vi "HFRR ADV v043.vi"() -> ()   [LabVIEW 2025] (continued)
            n814 = Subtract(x=w847, y=w851) -> (x-y=w855:dbl)
            n815 = In Range and Coerce(upper limit=w858, x=w850, lower limit=w857) -> (In Range?=w854:bool)  [unwired: 1 out]
            n816 = In Range and Coerce(upper limit=w856, x=w849, lower limit=w855) -> (In Range?=w853:bool)  [unwired: 1 out]
            n817 = And(x=w854, y=w853) -> (x .and. y?=w852:bool)
            n818 = case shown="True" w852 {
              frame False {
                n819 = property on="Accept & Save Air Temperature step 4" class="Bool (strict)"("DisabledEnum"=T19."Disabled" ("Disabled")) -> ()  [unwired: 2 in, 2 out]
                n820 = local write "Air Temperature Calibration"(enum32{"True", "Fail"}."Fail" ("Sample Temperature Calibration  2")) -> ()
              }
              frame True {
                n821 = local write "Air Temperature Calibration"(enum32{"True", "Fail"}."True" ("Sample Temperature Calibration  2")) -> ()
                n822 = property on="Accept & Save Air Temperature step 4" class="Bool (strict)"("DisabledEnum"=T19."Enabled" ("Disabled")) -> ()  [unwired: 2 in, 2 out]
              }
            }
          }
          frame #8 {
            # "CAL;END"
          }
          frame #9 {
            n823 = local write "Tab Control 4"(T12."Air Step 4" ("Tab Control 4")) -> ()
          }
        }
      }
      event "Back Stroke step main temperature": Value Change {
        n824 = event-data() -> ()  [unwired: 1 in, 6 out]
        n825 = stacked-sequence {
          frame #0 {
            n826 = Wait (ms)(milliseconds to wait=u32 1000) -> ()  [unwired: 1 out]
          }
          frame #1 {
            # "CAL;END"
            n827 = local write "Due Write"("CAL;END" ("Command")) -> ()
          }
          frame #2 {
            n828 = Wait (ms)(milliseconds to wait=u32 1000) -> ()  [unwired: 1 out]
          }
          frame #3 {
            # "CAL;END"
            n829 = local write "Due Write"("CAL;END" ("Command")) -> ()
          }
          frame #4 {
            n830 = local write "Temperature Selection"(T13."Default" ("Temperature Selection")) -> ()
            n831 = local write "Calibration Selection"(T8."Default" ("Calibration Selection")) -> ()
            n832 = local write "Main Calibration Tab"(T7."Main" ("Main Calibration Tab")) -> ()
            n833 = local write "Tab Control 4"(T12."Main" ("Tab Control 4")) -> ()
          }
        }
      }
      event "TEMPERATURE STEP  Back 4", "TEMPERATURE STEP 1 Back 3", "TEMPERATURE STEP  Back 3", "TEMPERATURE STEP 1 Back 2", "Back Air TEMPERATURE Step 4", "Back SAMPLE TEMPERATURE Step 4": Value Change {
        # "Back Stroke step main temperature"
        n834 = event-data() -> ()  [unwired: 1 in, 6 out]
        n835 = stacked-sequence {
          frame #0 {
            n836 = Wait (ms)(milliseconds to wait=u32 1000) -> ()  [unwired: 1 out]
          }
          frame #1 {
            # "CAL;END"
            n837 = local write "Due Write"("CAL;END" ("Command")) -> ()
          }
          frame #2 {
            n838 = Wait (ms)(milliseconds to wait=u32 1000) -> ()  [unwired: 1 out]
          }
          frame #3 {
            # "CAL;END"
            n839 = local write "Due Write"("CAL;END" ("Command")) -> ()
          }
          frame #4 {
            # "TEMPERATURE STEP  Back 4"
            n840 = local write "Main Calibration Tab"(T7."Temperature" ("Main Calibration Tab")) -> ()
            n841 = local write "Temperature Selection"(T13."Default" ("Temperature Selection")) -> ()
            n842 = local write "Tab Control 4"(T12."Main" ("Tab Control 4")) -> ()
            n843 = local write "Calibration Selection"(T8."Default" ("Calibration Selection")) -> ()
          }
        }
      }
      event "FF BACK", "FF BACK 2", "FF BACK 3", "FF BACK 4", "FF BACK 5", "FF BACK 6": Value Change {
        n844 = event-data() -> ()  [unwired: 1 in, 6 out]
        n845 = stacked-sequence {
          frame #0 {
            n846 = Wait (ms)(milliseconds to wait=u32 1000) -> ()  [unwired: 1 out]
          }
          frame #1 {
            n847 = local write "Due Write"("VC;0") -> ()
          }
          frame #2 {
            n848 = Wait (ms)(milliseconds to wait=u32 1000) -> ()  [unwired: 1 out]
          }
          frame #3 {
            n849 = local write "Due Write"("VC;0") -> ()
          }
          frame #4 {
            w884 = FALSE
            n850 = local write "FF BACK 2"(w884) -> ()
            n851 = local write "FF BACK 3"(w884) -> ()
            n852 = local write "FF BACK 4"(w884) -> ()
            n853 = local write "FF BACK 5"(w884) -> ()
            n854 = local write "FF BACK 6"(w884) -> ()
            n855 = local write "FF BACK"(w884) -> ()
          }
          frame #5 {
            n856 = local write "Temperature Selection"(T13."Default" ("Temperature Selection")) -> ()
            n857 = local write "Calibration Selection"(T8."Default" ("Calibration Selection")) -> ()
            n858 = local write "Friction Force Tab"(T11."Page 1" ("Friction Force Tab")) -> ()
            n859 = local write "Main Calibration Tab"(T7."Main" ("Main Calibration Tab")) -> ()
            n860 = property on="Tab Control 6" class="TabCtl (strict)"("Visible"=FALSE) -> ()  [unwired: 2 in, 2 out]
            n861 = property on="Friction Force Calibration Result Tab" class="TabCtl (strict)"("Visible"=FALSE) -> ()  [unwired: 2 in, 2 out]
          }
        }
      }
      event "Accept & Save FF": Value Change {
        n862 = event-data() -> ()  [unwired: 1 in, 6 out]
        n863 = stacked-sequence {
          frame #0 {
            n864 = Wait (ms)(milliseconds to wait=u32 1000) -> ()  [unwired: 1 out]
          }
          frame #1 {
            n865 = local write "Due Write"("VC;0") -> ()
          }
          frame #2 {
            n866 = Wait (ms)(milliseconds to wait=u32 1000) -> ()  [unwired: 1 out]
          }
          frame #3 {
            n867 = local write "Due Write"("VC;0") -> ()
          }
          frame #4 {
            w895 = FALSE
            n868 = local write "FF BACK 2"(w895) -> ()
            n869 = local write "FF BACK 3"(w895) -> ()
            n870 = local write "FF BACK 4"(w895) -> ()
            n871 = local write "FF BACK 5"(w895) -> ()
            n872 = local write "FF BACK 6"(w895) -> ()
            n873 = local write "FF BACK"(w895) -> ()
          }
          frame #5 {
            n874 = Get Date/Time In Seconds() -> (seconds since 1Jan1904=w898:timestamp)
            n875 = Format Into String(format string="%<%I:%M:%S:%p %d:%B:%Y>T", w898) -> (resulting string=w896:string)  [unwired: 2 in, 1 out]
            n876 = local write "FRICTION CALIBRATION"(w896) -> ()
          }
          frame #6 {
            n877 = local write "Temperature Selection"(T13."Default" ("Temperature Selection")) -> ()
            n878 = local write "Calibration Selection"(T8."Default" ("Calibration Selection")) -> ()
            n879 = local write "Friction Force Tab"(T11."Page 1" ("Friction Force Tab")) -> ()
            n880 = local write "Main Calibration Tab"(T7."Main" ("Main Calibration Tab")) -> ()
            n881 = local write "Save Button"(TRUE ("Save Button")) -> ()
            n882 = property on="Tab Control 6" class="TabCtl (strict)"("Visible"=FALSE) -> ()  [unwired: 2 in, 2 out]
            n883 = property on="Friction Force Calibration Result Tab" class="TabCtl (strict)"("Visible"=FALSE) -> ()  [unwired: 2 in, 2 out]
          }
        }
      }
      event "FF CONTINUE": Value Change {
        n884 = event-data() -> ()  [unwired: 1 in, 6 out]
        n885 = local write "FF CONTINUE"(FALSE ("FF CONTINUE")) -> ()
        n886 = local write "Friction Force Tab"(T11."Page 2" ("Friction Force Tab")) -> ()
      }
      event "FF CONTINUE 2": Value Change {
        n887 = event-data() -> ()  [unwired: 1 in, 6 out]
        n888 = local write "FF CONTINUE 2"(FALSE ("FF CONTINUE")) -> ()
        n889 = local write "Friction Force Tab"(T11."Page 3" ("Friction Force Tab")) -> ()
      }
      event "FF CONTINUE 3": Value Change {
        n890 = event-data() -> ()  [unwired: 1 in, 6 out]
        n891 = local write "FF CONTINUE 3"(FALSE ("FF CONTINUE")) -> ()
        n892 = local write "Friction Force Tab"(T11."Page 4" ("Friction Force Tab")) -> ()
      }
      event "FF CONTINUE 4": Value Change {
        n893 = event-data() -> ()  [unwired: 1 in, 6 out]
        n894 = local write "FF CONTINUE 4"(FALSE ("FF CONTINUE")) -> ()
        n895 = local write "Friction Force Tab"(T11."Page 5" ("Friction Force Tab")) -> ()
        n896 = property on="Friction Force Calibration Result Tab" class="TabCtl (strict)"("Visible"=FALSE) -> ()  [unwired: 2 in, 2 out]
      }
      event "FF CONTINUE 5": Value Change {
        n897 = event-data() -> ()  [unwired: 1 in, 6 out]
        n898 = local write "FF CONTINUE 5"(FALSE ("FF CONTINUE")) -> ()
        n899 = local write "Friction Force Tab"(T11."Page 6" ("Friction Force Tab")) -> ()
        n900 = property on="Friction Force Calibration Result Tab" class="TabCtl (strict)"("Visible"=FALSE) -> ()  [unwired: 2 in, 2 out]
        n901 = property on="Tab Control 6" class="TabCtl (strict)"("Visible"=FALSE) -> ()  [unwired: 2 in, 2 out]
      }
      event "Stroke Report Button": Value Change {
        n902 = event-data() -> ()  [unwired: 1 in, 6 out]
        n903 = local read "Point 5 - 1.0 mm"() -> (w920:bool)
        n904 = case shown="False" w920 {
          tunnel: [0.8 1.0] -> w919
          frame False {
          }
          frame True {
          }
        }
        n905 = local read "Machine Serial Number"() -> (w923:string)
        n906 = local read "USERNAME"() -> (w921:string)
        n907 = local write "Stroke Report Button"(FALSE ("Stroke Report Button")) -> ()
        n908 = call "Stroke Calibration Report.vi"("measured_value"=w919, "operator_name"=w921, "Instrument_serial Number"=w923) -> ()  [unwired: 7 in, 2 out]
      }
      event "Sample Report Button": Value Change {
        n909 = event-data() -> ()  [unwired: 1 in, 6 out]
        n910 = local read "Machine Serial Number"() -> (w929:string)
        n911 = local read "Sample 0deg temp"() -> (w926:dbl)
        n912 = local read "Sample 60deg temp"() -> (w927:dbl)
        n913 = local read "USERNAME"() -> (w928:string)
        n914 = call "Temperature Calibration Report.vi"("measured_60"=w927, "measured_zero"=w926, "operator_name"=w928, "Instrument_serial Number"=w929) -> ()  [unwired: 6 in, 2 out]
        n915 = local write "Sample Report Button"(FALSE ("Sample Report Button")) -> ()
      }
      event "Report Button FF": Value Change {
        n916 = event-data() -> ()  [unwired: 1 in, 6 out]
        n917 = local read "FF PASS"() -> (w934:bool)
        n918 = local read "Machine Serial Number"() -> (w937:string)
        n919 = Select(t="PASS", s=w934, f="FAIL") -> (s? t:f=w931:string)
        n920 = local read "USERNAME"() -> (w936:string)
        n921 = call "FF Calibration Report.vi"("pass_or_fail"=w931, "operator_name"=w936, "Instrument_serial Number"=w937) -> ()  [unwired: 7 in, 2 out]
        n922 = local write "Report Button FF"(FALSE ("Sample Report Button")) -> ()
      }
      event "Air Temperature Report Button": Value Change {
        n923 = event-data() -> ()  [unwired: 1 in, 6 out]
        n924 = local read "Machine Serial Number"() -> (w942:string)
        n925 = local read "Air 0deg temp"() -> (w939:dbl)
        n926 = local read "Air 60deg temp"() -> (w940:dbl)
        n927 = local read "USERNAME"() -> (w941:string)
        n928 = call "Air Temperature Calibration Report.vi"("measured_60"=w940, "measured_zero"=w939, "operator_name"=w941, "Instrument_serial Number"=w942) -> ()  [unwired: 6 in, 2 out]
        n929 = local write "Air Temperature Report Button"(FALSE ("Sample Report Button")) -> ()
      }
      event "Quit": Value Change {
        n930 = event-data() -> ()  [unwired: 1 in, 6 out]
      }
    }
    n931 = Wait (ms)(milliseconds to wait=u32 100) -> ()  [unwired: 1 out]
  }
  n932 = while {
    shift-right: [w945] -> _
    shift-left: "Enum - Selector" -> [w946]
    stop <- w947 stop-if-true
    # "Auto Start Logic Loop"
    n933 = case shown="\"Maintain Stage\"" w946 {
      tunnel: [w950 w956 w984 w1019 w1049 Auto_Start_enum."Exit" ("Enum - Selector") Auto_Start_enum."Init" ("Enum - Selector")] -> w945
      frame "Init", Default {
        n934 = local read "Auto Start Test"() -> (w949:bool)
        n935 = Select(t=Auto_Start_enum."Humidity & Temperature On" ("Enum - Selector"), s=w949, f=Auto_Start_enum."Init") -> (s? t:f=w950:T15)
      }
      frame "Humidity & Temperature On" {
        n936 = stacked-sequence {
          tunnel: [_ _ _ _ _ _ Auto_Start_enum."Reach point" ("Enum - Selector")] -> w953
          frame #0 {
            w958 = T19."Disabled and Grayed Out" ("Disabled")
            w959 = TRUE ("Heater Button")
            n937 = property on="Humidity" class="Bool (strict)"("DisabledEnum"=w958) -> ()  [unwired: 2 in, 2 out]
            n938 = property on="Heater Button" class="Bool (strict)"("DisabledEnum"=w958) -> ()  [unwired: 2 in, 2 out]
            n939 = local write "Heater Button"(w959) -> ()
            n940 = local write "Humidity"(w959) -> ()
            n941 = property on="Heater Button" class="Bool (strict)"("Val(Sgnl)"=TRUE ("Value (Signaling)")) -> ()  [unwired: 2 in, 2 out]
          }
          frame #1 {
            n942 = Wait (ms)(milliseconds to wait=u32 3000) -> ()  [unwired: 1 out]
          }
          frame #2 {
            n943 = local read "Set Temp"() -> (w965:dbl)
            n944 = Number To Fractional String(number=w965, precision (6)=i16 2) -> (F-format string=w962:string)  [unwired: 2 in]
            n945 = Concatenate Strings("ST;" ("Command"), w962) -> (w963:string)
            n946 = local write "Due Write"(w963) -> ()
          }
          frame #3 {
            n947 = Wait (ms)(milliseconds to wait=u32 1500) -> ()  [unwired: 1 out]
          }
          frame #4 {
            (unwired) i16 2 ("precision (6)")
            n948 = local read "WriteHumidity"() -> (w967:string[])
            n949 = local read "Set Rh"() -> (w970:dbl)
            n950 = Number To Fractional String(number=w970) -> (F-format string=w971:string)  [unwired: 3 in]
            n951 = Concatenate Strings("M;" ("new element/subarray"), w971) -> (w972:string)
            n952 = Insert Into Array(array=w967, new element=w972) -> (w968:string[])  [unwired: 1 in]
            n953 = local write "WriteHumidity"(w968) -> ()
            n954 = local write "Due Write"("HE;1" ("Command")) -> ()
          }
          frame #5 {
            n955 = Wait (ms)(milliseconds to wait=u32 1500) -> ()  [unwired: 1 out]
          }
          frame #6 {
            w975 = TRUE ("Reach point temp")
            n956 = local write "Reach point Humidity"(w975) -> ()
            n957 = local write "Reach point temp"(w975) -> ()
          }
        }
        n958 = local read "Auto Start Test"() -> (w955:bool)
        n959 = Not(x=w955) -> (.not. x?=w954:bool)
        n960 = Select(t=Auto_Start_enum."close", s=w954, f=w953) -> (s? t:f=w956:T15)
      }
      frame "Reach point" {
        w985 = TRUE ("PAUSE")
        w993 = 1.0 ("y")
        w996 = 1.0 ("y")
        n961 = local read "Set Temp"() -> (w978:dbl)
        n962 = local read "Set Humidity:"() -> (w992:dbl)
        n963 = local read "Humidity ( %RH )"() -> (w997:dbl)
        n964 = Add(x=w978, y=w996) -> (x+y=w995:dbl)
        n965 = Subtract(x=w978, y=w996) -> (x-y=w994:dbl)
        n966 = Add(x=w992, y=w993) -> (x+y=w991:dbl)
        n967 = Subtract(x=w992, y=w993) -> (x-y=w990:dbl)
        n968 = local read "TEMP"() -> (w998:dbl)
        n969 = In Range and Coerce(upper limit=w991, x=w997, lower limit=w990) -> (In Range?=w979:bool)  [unwired: 1 out]
        n970 = In Range and Coerce(upper limit=w995, x=w998, lower limit=w994) -> (In Range?=w980:bool)  [unwired: 1 out]
        n971 = disable-structure shown="Enabled" {
          disable-tunnel: w979 -> [w999 _]
          disable-tunnel: [w999 TRUE] -> w977
          frame Disabled {
            n972 = case shown="True" w999 {
              frame False {
              }
              frame True {
                n973 = case shown="True" "Reach point Humidity" {
                  selector: "Reach point Humidity" -> [_ w1005]
                  frame False {
                  }
                  frame True {
                    n974 = local read "EVENT LOG"() -> (w1002:string)
                    n975 = Not(x=w1005) -> (.not. x?=w1004:bool)
                    n976 = local write "Reach point Humidity"(w1004) -> ()
                    n977 = call "Event Log.vi"("Content"="Target Humidity reached", "EVENT LOG"=w1002) -> ("EVENT LOG"=w1003:string)  [unwired: 8 in, 1 out]
                    n978 = local write "EVENT LOG"(w1003) -> ()
                  }
                }
              }
            }
          }
          frame Enabled {
          }
        }
        n979 = case shown="True" w980 {
          frame False {
          }
          frame True {
            n980 = case shown="True" "Reach point temp" {
              selector: "Reach point temp" -> [_ w1012]
              frame False {
              }
              frame True {
                n981 = local read "EVENT LOG"() -> (w1009:string)
                n982 = Not(x=w1012) -> (.not. x?=w1011:bool)
                n983 = local write "Reach point temp"(w1011) -> ()
                n984 = call "Event Log.vi"("Content"="Target Temperature reached", "EVENT LOG"=w1009) -> ("EVENT LOG"=w1010:string)  [unwired: 8 in, 1 out]
                n985 = local write "EVENT LOG"(w1010) -> ()
              }
            }
          }
        }
        n986 = local read "Auto Start Test"() -> (w983:bool)
        n987 = And(x=w980, y=w977) -> (x .and. y?=w989:bool)
        n988 = Select(t=Auto_Start_enum."Maintain Stage" ("Enum - Selector"), s=w989, f=Auto_Start_enum."Reach point" ("Enum - Selector")) -> (s? t:f=w986:T15)
        n989 = Not(x=w983) -> (.not. x?=w982:bool)
        n990 = Select(t=Auto_Start_enum."close", s=w982, f=w986) -> (s? t:f=w984:T15)
        n991 = call "ELAPSED TIMER VI.vi"("RESET"=w985, "PAUSE"=w985) -> ()  [unwired: 7 in, 3 out]
      }
      frame "Maintain Stage" {
        w1027 = 2.0 ("y")
        w1026 = 1.0 ("y")
        # "Humidity and temperature set point has stabilized."
        # "Humidity and  temperatures Set Point  have been reached"
        n992 = local read "Set Temp"() -> (w1014:dbl)
        n993 = local read "Set Humidity:"() -> (w1030:dbl)
        n994 = local read "Humidity ( %RH )"() -> (w1033:dbl)
        n995 = Add(x=w1014, y=w1026) -> (x+y=w1032:dbl)
        n996 = Subtract(x=w1014, y=w1026) -> (x-y=w1031:dbl)
        n997 = local read "TEMP"() -> (w1034:dbl)
        n998 = Add(x=w1030, y=w1027) -> (x+y=w1029:dbl)
        n999 = Subtract(x=w1030, y=w1027) -> (x-y=w1028:dbl)
        n1000 = In Range and Coerce(upper limit=w1032, x=w1034, lower limit=w1031) -> (In Range?=w1025:bool)  [unwired: 1 out]
        n1001 = In Range and Coerce(upper limit=w1029, x=w1033, lower limit=w1028) -> ()  [unwired: 2 out]
        n1002 = And(x=w1025, y=TRUE) -> (x .and. y?=w1024:bool)
        n1003 = Not(x=w1024) -> (.not. x?=w1023:bool)
        n1004 = call "ELAPSED TIMER VI.vi"("TARGET"=60.0, "RESET"=w1023, "PAUSE"=FALSE) -> ("ELAPSED INDICATION"=w1020:bool)  [unwired: 6 in, 2 out]
        n1005 = case shown="True" w1020 {
          tunnel: w1020 -> [_ w1037]
          tunnel: [Auto_Start_enum."Maintain Stage" ("Enum - Selector") w1036] -> w1018
          frame False {
          }
          frame True {
            n1006 = stacked-sequence {
              tunnel: w1037 -> [_ _ _ _ _]
              tunnel: [_ _ _ _ Auto_Start_enum."Start Stage" ("Enum - Selector")] -> w1036
              frame #0 {
                n1007 = local read "EVENT LOG"() -> (w1039:string)
                n1008 = call "Event Log.vi"("Content"="Temperature set point has stabilized.", "EVENT LOG"=w1039) -> ("EVENT LOG"=w1040:string)  [unwired: 8 in, 1 out]
                n1009 = local write "EVENT LOG"(w1040) -> ()
              }
              frame #1 {
                n1010 = Wait (ms)(milliseconds to wait=u32 100) -> ()  [unwired: 1 out]
              }
              frame #2 {
                n1011 = local read "EVENT LOG"() -> (w1044:string)
                n1012 = call "Event Log.vi"("Content"="Auto Test Started", "EVENT LOG"=w1044) -> ("EVENT LOG"=w1045:string)  [unwired: 8 in, 1 out]
                n1013 = local write "EVENT LOG"(w1045) -> ()
                n1014 = local write "FRICVALZ 4"(TRUE ("FRICVALZ 4")) -> ()
              }
              frame #3 {
                w1046 = TRUE ("RUN")
                n1015 = local write "RUN"(w1046) -> ()
                n1016 = property on="Auto Start Temp" class="Bool (strict)"("Val(Sgnl)"=w1046) -> ()  [unwired: 2 in, 2 out]
                "Auto Start Temp" <- w1046
              }
              frame #4 {
              }
            }
          }
        }
        n1017 = local read "Auto Start Test"() -> (w1017:bool)
        n1018 = Not(x=w1017) -> (.not. x?=w1016:bool)
        n1019 = Select(t=Auto_Start_enum."close", s=w1016, f=w1018) -> (s? t:f=w1019:T15)
      }
      frame "Start Stage" {
        w1048 = TRUE ("PAUSE")
        n1020 = local read "Auto Start Test"() -> (w1053:bool)
        n1021 = Not(x=w1053) -> (.not. x?=w1052:bool)
        n1022 = Select(t=Auto_Start_enum."close" ("Enum - Selector"), s=w1052, f=Auto_Start_enum."Start Stage" ("Enum - Selector")) -> (s? t:f=w1049:T15)
        n1023 = call "ELAPSED TIMER VI.vi"("RESET"=w1048, "PAUSE"=w1048) -> ()  [unwired: 7 in, 3 out]
      }
      frame "close" {
        w1056 = FALSE ("Heater Button")
        n1024 = local write "RUN"(w1056) -> ()
        n1025 = local write "Heater Button"(w1056) -> ()
        n1026 = local write "Humidity"(w1056) -> ()
        n1027 = local write "Auto Start Test"(w1056) -> ()
        n1028 = property on="Heater Button" class="Bool (strict)"("Val(Sgnl)"=FALSE ("Value (Signaling)")) -> ()  [unwired: 2 in, 2 out]
        n1029 = local write "Humidity 2"(TRUE ("Humidity")) -> ()
      }
      frame "Exit" {
      }
    }
    n1030 = Wait (ms)(milliseconds to wait=u32 100) -> ()  [unwired: 1 out]
    n1031 = local read "Quit"() -> (w947:bool)
  }
  n1032 = property on="Service Password Log" class="Str"("Visible"=w25) -> ()  [unwired: 2 in, 2 out]
  n1033 = property on="Password 3" class="Clust (strict)"("Visible"=w25) -> ()  [unwired: 2 in, 2 out]
  n1034 = while {
    stop <- w1085 stop-if-true
    w1068 = errorcluster {"status"=FALSE, "code"=0, "source"=""} ("error in (no error) 3")
    # "this loop is for manual report generation"
    n1035 = local read "Confirm Measrurement"() -> (w1067:bool)
    n1036 = case shown="True" w1067 {
      selector: w1067 -> [_ w1175]
      tunnel: errorcluster {"status"=FALSE, "code"=0, "source"=""} ("error in (no error) 3") -> [_ w1176]
      tunnel: [_ w1174] -> _
      frame False {
      }
      frame True {
        n1037 = stacked-sequence {
          tunnel: w1176 -> [_ w1209 _]
          tunnel: w1175 -> [_ _ w1316]
          tunnel: [_ w1197 _] -> w1174
          frame #0 {
            n1038 = String To Path(string="C:\\LAB-IQ\\Image Calibrate v01.dcf") -> (path=w1179:path)
            n1039 = Open/Create/Replace File ("Open File")(file path (use dialog)=w1179) -> (refnum out=w1180:refnum<file>)  [unwired: 5 in, 2 out]
            n1040 = for {
              N: 4 -> [_]
              tunnel: w1180 -> [w1186]
              i -> [w1182]
              n1041 = Read from Text File ("Read File")(file (use dialog)=w1186) -> (text=w1187:string)  [unwired: 3 in, 3 out]
              n1042 = String Subset(string=w1187, offset (0)=6, length (rest)=10 ("length (rest)")) -> (substring=w1183:string)
              n1043 = Fract/Exp String To Number(string=w1183) -> (number=w1181:dbl)  [unwired: 3 in, 1 out]
              n1044 = case shown="3" w1182 {
                tunnel: w1181 -> [w1188 w1189 _ w1190 _]
                frame 0 {
                  n1045 = local write "5x Gain"(w1188) -> ()
                }
                frame 1 {
                  n1046 = local write "10x Gain"(w1189) -> ()
                }
                frame 2 {
                }
                frame 3 {
                  n1047 = local write "100x gain"(w1190) -> ()
                }
                frame 4, Default {
                }
              }
            }
          }
          frame #1 {
            n1048 = local read "TEST STANDARD"() -> (w1192:T3)
            n1049 = case shown="\"ISO 12156\"" w1192 {
              tunnel: ["ASTM D6079" "ISO 12156"] -> w1191
              frame "ASTM D6079", Default {
              }
              frame "ISO 12156" {
              }
            }
            n1050 = call "IMAGE ANALYSIS.vi"("Enum"=POST_ANALYSIS_ENUM."GET MEASUREMENTS", "error in"=w1209) -> ("error out"=w1216:errorcluster)  [unwired: 8 in, 1 out]
            n1051 = local read "Magnification :"() -> (w1202:string)
            n1052 = call "Stall Data Flow.vim"("value in"=w1216, "milliseconds to wait"=u32 1000) -> ("value out"=w1215:errorcluster)  [unwired: 1 out]
            n1053 = local read "Test File List :"() -> (w1213:string)
            n1054 = case shown="\"10x\"" w1202 {
              tunnel: [w1252 w1253] -> w1200
              frame "5x", Default {
                n1055 = local read "5x Gain"() -> (w1252:dbl)
              }
              frame "10x" {
                # "5x"
                n1056 = local read "10x Gain"() -> (w1253:dbl)
              }
            }
            n1057 = call "IMAGE ANALYSIS.vi"("Enum"=POST_ANALYSIS_ENUM."READ", "error in"=w1215) -> ("error out"=w1212:errorcluster, "data out"=w1203:string)  [unwired: 8 in]
            n1058 = Match Pattern(string=w1203, regular expression="\"type\": ") -> (after substring=w1207:string)  [unwired: 1 in, 3 out]
            n1059 = call "IMAGE PATH CREATION PY.vi"("error in (no error)"=w1212, "File Name :"=w1213) -> ("error out"=w1211:errorcluster, "File Path"=w1199:path, "File Path String:"=w1194:string)  [unwired: 7 in]
            n1060 = Match Pattern(string=w1207, regular expression=",") -> (before substring=w1193:string)  [unwired: 1 in, 3 out]
            n1061 = local read "Calibration Tab"() -> (w1196:enum32{"Measrument", "Calibrate"})
            n1062 = call "Stall Data Flow.vim"("value in"=w1211, "milliseconds to wait"=u32 250) -> ("value out"=w1195:errorcluster)  [unwired: 1 out]
            n1063 = Equal?(x=w1193, y="\"rectangle\"") -> (x = y?=w1204:bool)
            n1064 = case shown="False" w1204 {
              tunnel: w1203 -> [w1258 w1313]
              tunnel: w1200 -> [_ w1304]
              tunnel: cluster{"major":dbl, "minor":dbl, "average":dbl} {"major"=0.0, "minor"=0.0, "average"=0.0} -> [w1256 w1300]
              tunnel: [w1255 w1297] -> w1198
              tunnel: w1193 -> [w1257 _]
              tunnel: w1200 -> [w1254 _]
              frame False {
                n1065 = Equal?(x=w1257, y="\"line\"") -> (x = y?=w1259:bool)
                n1066 = case shown="True" w1259 {
                  tunnel: w1258 -> [_ w1274]
                  tunnel: w1256 -> [w1261 w1273]
                  tunnel: [w1261 w1271] -> w1255
                  tunnel: w1254 -> [_ w1270]
                  frame False {
                  }
                  frame True {
                    w1269 = 0.0 ("Major Axis")
                    n1067 = Match Pattern(string=w1274, regular expression="\"length_px\":") -> (after substring=w1272:string)  [unwired: 1 in, 3 out]
                    n1068 = property on="Major Axis" class="DigNum (strict)"("Caption.Text"="") -> ()  [unwired: 2 in, 2 out]
                    n1069 = property on="Minor Axis" class="DigNum (strict)"("Caption.Text"="") -> ()  [unwired: 2 in, 2 out]
                    n1070 = property on="Average" class="DigNum (strict)"("Caption.Text"="Line") -> ()  [unwired: 2 in, 2 out]
                    n1071 = Fract/Exp String To Number(string=w1272, default (0 dbl)=0.0 ("default (0 DBL)")) -> (number=w1268:dbl)  [unwired: 2 in, 1 out]
                    "Pixel Value" <- w1268
                    n1072 = Multiply(x=w1268, y=w1270) -> (x*y=w1281:dbl)
                    n1073 = Multiply(x=w1281, y=1000.0) -> (x*y=w1264:dbl)
                    n1074 = Divide(x=w1264, y=1000.0) -> (x/y=w1267:dbl)
                    n1075 = local write "Measurment (mm)"(w1267) -> ()
                    n1076 = Bundle By Name(cluster=w1273, "average"=w1264) -> (w1271:cluster{"major":dbl, "minor":dbl, "average":dbl})
                    n1077 = Number To Fractional String(number=w1264, precision (6)=i16 1) -> (F-format string=w1263:string)  [unwired: 2 in]
                    n1078 = local write "Minor Axis"(w1269) -> ()
                    n1079 = local write "Major Axis"(w1269) -> ()
                    n1080 = Fract/Exp String To Number(string=w1263) -> (number=w1262:dbl)  [unwired: 3 in, 1 out]
                    n1081 = local write "Average"(w1262) -> ()
                  }
                }
              }
              frame True {
                w1301 = 1000.0 ("y")
                w1307 = 0.0 ("default (0 DBL)")
                n1082 = Match Pattern(string=w1313, regular expression=" \"width_px\":") -> (after substring=w1311:string)  [unwired: 1 in, 3 out]
                n1083 = Match Pattern(string=w1311, regular expression="\"height_px\":") -> (before substring=w1309:string, after substring=w1308:string)  [unwired: 1 in, 2 out]
                n1084 = Fract/Exp String To Number(string=w1309, default (0 dbl)=w1307) -> (number=w1306:dbl)  [unwired: 2 in, 1 out]
                n1085 = Fract/Exp String To Number(string=w1308, default (0 dbl)=w1307) -> (number=w1305:dbl)  [unwired: 2 in, 1 out]
                n1086 = Multiply(x=w1306, y=w1304) -> (x*y=w1303:dbl)
                n1087 = Multiply(x=w1305, y=w1304) -> (x*y=w1302:dbl)
                n1088 = Multiply(x=w1303, y=w1301) -> (x*y=w1287:dbl)
                n1089 = Multiply(x=w1302, y=w1301) -> (x*y=w1285:dbl)
                n1090 = Add(x=w1287, y=w1285) -> (x+y=w1299:dbl)
                n1091 = property on="Major Axis" class="DigNum (strict)"("Caption.Text"="Major Axis") -> ()  [unwired: 2 in, 2 out]
                n1092 = property on="Minor Axis" class="DigNum (strict)"("Caption.Text"="Minor Axis") -> ()  [unwired: 2 in, 2 out]
                n1093 = property on="Average" class="DigNum (strict)"("Caption.Text"="Average") -> ()  [unwired: 2 in, 2 out]
                n1094 = Divide(x=w1299, y=2.0) -> (x/y=w1283:dbl)
                n1095 = Bundle By Name(cluster=w1300, "major"=w1287, "minor"=w1285, "average"=w1283) -> (w1297:cluster{"major":dbl, "minor":dbl, "average":dbl})
                n1096 = Number To Fractional String(number=w1285, precision (6)=i16 1) -> (F-format string=w1292:string)  [unwired: 2 in]
                n1097 = Number To Fractional String(number=w1283, precision (6)=i16 1) -> (F-format string=w1293:string)  [unwired: 2 in]
                n1098 = Number To Fractional String(number=w1287, precision (6)=i16 1) -> (F-format string=w1291:string)  [unwired: 2 in]
                n1099 = Fract/Exp String To Number(string=w1292) -> (number=w1284:dbl)  [unwired: 3 in, 1 out]
                n1100 = Fract/Exp String To Number(string=w1293) -> (number=w1282:dbl)  [unwired: 3 in, 1 out]
                n1101 = Fract/Exp String To Number(string=w1291) -> (number=w1286:dbl)  [unwired: 3 in, 1 out]
                n1102 = local write "Major Axis"(w1286) -> ()
                n1103 = local write "Average"(w1282) -> ()
                n1104 = local write "Minor Axis"(w1284) -> ()
              }
            }
            n1105 = case shown="\"Measrument\", Default" w1196 {
              tunnel: w1199 -> [w1226 _]
              tunnel: w1198 -> [w1225 _]
              tunnel: [w1222 w1251] -> w1197
              tunnel: w1195 -> [w1224 w1251]
              tunnel: w1194 -> [w1223 _]
              tunnel: w1191 -> [w1221 _]
              frame "Measrument", Default {
                n1106 = stacked-sequence {
                  tunnel: w1226 -> [w1244 _]
                  tunnel: w1225 -> [w1242 _]
                  tunnel: w1224 -> [w1240 _]
                  tunnel: w1223 -> [w1239 _]
                  tunnel: [w1234 _] -> w1222
                  tunnel: w1221 -> [w1227 _]
                  frame #0 {
                    n1107 = call "IMAGE ANALYSIS.vi"("Enum"=POST_ANALYSIS_ENUM."SAVE IMAGE", "error in"=w1240, "IMAGE FILE PATH"=w1239) -> ("error out"=w1238:errorcluster)  [unwired: 7 in, 1 out]
                    n1108 = call "Stall Data Flow.vim"("value in"=w1238, "milliseconds to wait"=u32 1000) -> ("value out"=w1229:errorcluster)  [unwired: 1 out]
                    n1109 = local read "Test File List :"() -> (w1246:string)
                    n1110 = call "IMAGE ANALYSIS.vi"("Enum"=POST_ANALYSIS_ENUM."MINIMIZE UI", "error in"=w1229) -> ("error out"=w1236:errorcluster)  [unwired: 8 in, 1 out]
                    n1111 = Bundle By Name(cluster=T26 {"File Name"="", "Test Method"="", "Operator"="", "Fuel Description"="", "Date and time"=""} ("Main Ref"), "Test Method"=w1227, "File Name"=w1246) -> (w1247:T26)
                    n1112 = call "Stall Data Flow.vim"("value in"=w1236, "milliseconds to wait"=u32 1500) -> ("value out"=w1231:errorcluster)  [unwired: 1 out]
                    n1113 = call "duf file read.vi"("error in (no error)"=w1231, "Main Ref"=w1247) -> ("error out"=w1245:errorcluster, "Main Ref 2"=w1243:T26)  [unwired: 8 in]
                    n1114 = call "DETECTION REPORT for manual.vi"("error in (no error)"=w1245, "return value 3"=w1242, "Image File Path"=w1244, "Main Ref"=w1243) -> ("error out"=w1241:errorcluster)  [unwired: 7 in]
                    n1115 = call <vilib>:"Clear Errors.vi"("error in (no error)"=w1241) -> ("error out"=w1232:errorcluster)  [unwired: 5 in, 1 out]
                    n1116 = call "IMAGE ANALYSIS.vi"("Enum"=POST_ANALYSIS_ENUM."MINIMIZE UI", "error in"=w1232) -> ("error out"=w1234:errorcluster)  [unwired: 8 in, 1 out]
                  }
                  frame #1 {
                    n1117 = local write "Main Tab"(T2."HOME" ("Main Tab")) -> ()
                    n1118 = local write "Main Dashboard Buttons"(T1."Home" ("Main Dashboard Buttons")) -> ()
                  }
                }
              }
              frame "Calibrate" {
              }
            }
          }
          frame #2 {
            n1119 = Not(x=w1316) -> (.not. x?=w1315:bool)
            n1120 = local write "Confirm Measrurement"(w1315) -> ()
            n1121 = local read "Calibration Tab"() -> (w1314:enum32{"Measrument", "Calibrate"})
            n1122 = case shown="\"Measrument\", Default" w1314 {
              frame "Measrument", Default {
                (unwired) T21."HOME" ("Main Tab")
                n1123 = local write "Main Tab"(T2."HOME" ("Main Tab")) -> ()
              }
              frame "Calibrate" {
              }
            }
          }
        }
      }
    }
    n1124 = local read "Humidity"() -> (w1059:bool)
    n1125 = local read "Save Change"() -> (w1064:bool)
    n1126 = local read "Calibrate"() -> (w1065:bool)
    n1127 = local read "Auto Start Test"() -> (w1060:bool)
    n1128 = case shown="True" w1065 {
      selector: w1065 -> [_ w1172]
      frame False {
      }
      frame True {
        n1129 = Not(x=w1172) -> (.not. x?=w1171:bool)
        n1130 = local write "Calibrate"(w1171) -> ()
        n1131 = local write "Calibration Tab"(enum32{"Measrument", "Calibrate"}."Calibrate" ("Calibration Tab")) -> ()
      }
    }
    n1132 = case shown="True" w1064 {
      selector: w1064 -> [_ w1116]
      frame False {
      }
      frame True {
        n1133 = stacked-sequence {
          tunnel: w1116 -> [_ _ _ _ w1170]
          frame #0 {
            n1134 = call "IMAGE ANALYSIS.vi"("Enum"=POST_ANALYSIS_ENUM."HIDE UI") -> ()  [unwired: 9 in, 2 out]
          }
          frame #1 {
            n1135 = local read "100x gain"() -> (w1118:dbl)
            n1136 = local read "10x Gain"() -> (w1119:dbl)
            n1137 = local read "5x Gain"() -> (w1120:dbl)
            n1138 = Number To Fractional String(number=w1119, width (-)=i16 4, precision (6)=i16 7) -> (F-format string=w1141:string)  [unwired: 1 in]
            n1139 = Number To Fractional String(number=0.0, width (-)=i16 4, precision (6)=i16 7) -> (F-format string=w1136:string)  [unwired: 1 in]
            n1140 = Number To Fractional String(number=w1118, width (-)=i16 4, precision (6)=i16 7) -> (F-format string=w1124:string)  [unwired: 1 in]
            n1141 = Number To Fractional String(number=w1120, width (-)=i16 10 ("precision (6)"), precision (6)=i16 7) -> (F-format string=w1150:string)  [unwired: 1 in]
            n1142 = Concatenate Strings("[CH1]" ("string"), w1150, " - 5x Gain" ("string"), "\r") -> (w1140:string)
            n1143 = Concatenate Strings("[CH2]" ("string"), w1141, " - 10x Gain" ("string"), "\r") -> (w1139:string)
            n1144 = Concatenate Strings("[CH3]" ("string"), w1136, " - 20x Gain" ("string"), "\r") -> (w1130:string)
            n1145 = Concatenate Strings("[CH4]" ("string"), w1124, " - 100x Gain" ("string"), "\r") -> (w1123:string)
            n1146 = String To Path(string="C:\\LAB-IQ\\Image Calibrate v01.dcf") -> (path=w1153:path)
            n1147 = Concatenate Strings(w1140, w1139, w1130, w1123) -> (w1138:string)
            n1148 = call <vilib>:"Write Characters To File.vi"("append to file? (new file:F)"=FALSE, "character string"=w1138, "file path (dialog if empty)"=w1153) -> ()  [unwired: 2 in, 1 out]
          }
          frame #2 {
            n1149 = String To Path(string="C:\\LAB-IQ\\Image Calibrate v01.dcf") -> (path=w1156:path)
            n1150 = Open/Create/Replace File ("Open File")(file path (use dialog)=w1156) -> (refnum out=w1157:refnum<file>)  [unwired: 5 in, 2 out]
            n1151 = for {
              N: 4 -> [_]
              tunnel: w1157 -> [w1163]
              i -> [w1159]
              n1152 = Read from Text File ("Read File")(file (use dialog)=w1163) -> (text=w1164:string)  [unwired: 3 in, 3 out]
              n1153 = String Subset(string=w1164, offset (0)=6, length (rest)=10 ("length (rest)")) -> (substring=w1160:string)
              n1154 = Fract/Exp String To Number(string=w1160) -> (number=w1158:dbl)  [unwired: 3 in, 1 out]
              n1155 = case shown="3" w1159 {
                tunnel: w1158 -> [w1165 w1166 _ w1167 _]
                frame 0 {
                  n1156 = local write "5x Gain"(w1165) -> ()
                }
                frame 1 {
                  n1157 = local write "10x Gain"(w1166) -> ()
                }
                frame 2 {
                }
                frame 3 {
                  n1158 = local write "100x gain"(w1167) -> ()
                }
                frame 4, Default {
                }
              }
            }
          }
          frame #3 {
            n1159 = call "IMAGE ANALYSIS.vi"("Enum"=POST_ANALYSIS_ENUM."SHOW UI") -> ()  [unwired: 9 in, 2 out]
          }
          frame #4 {
            n1160 = Not(x=w1170) -> (.not. x?=w1169:bool)
            n1161 = local write "Save Change"(w1169) -> ()
          }
        }
      }
    }
    n1162 = case shown="False" w1060 {
      tunnel: w1059 -> [w1086 _]
      frame False {
        n1163 = case shown="True" w1086 {
          frame False {
          }
          frame True {
            n1164 = local read "Set Humidity:"() -> (w1090:dbl)
            n1165 = local read "Set Humidity:"() -> (w1093:dbl)
            n1166 = local read "Humidity ( %RH )"() -> (w1094:dbl)
            n1167 = Subtract(x=w1090, y=2.0) -> (x-y=w1088:dbl)
            n1168 = Add(x=w1093, y=2.0) -> (x+y=w1089:dbl)
            n1169 = In Range and Coerce(upper limit=w1089, x=w1094, lower limit=w1088) -> (In Range?=w1087:bool)  [unwired: 1 out]
            n1170 = case shown="True" w1087 {
              frame False {
              }
              frame True {
                n1171 = case shown="True" "Manual Humididty Reached" {
                  selector: "Manual Humididty Reached" -> [_ w1097]
                  frame False {
                  }
                  frame True {
                    n1172 = Not(x=w1097) -> (.not. x?=w1096:bool)
                    n1173 = local write "Manual Humididty Reached"(w1096) -> ()
                    n1174 = local read "EVENT LOG"() -> (w1099:string)
                    n1175 = call "Event Log.vi"("Content"="Target Humidity reached", "EVENT LOG"=w1099) -> ("EVENT LOG"=w1098:string)  [unwired: 8 in, 1 out]
                    n1176 = local write "EVENT LOG"(w1098) -> ()
                  }
                }
              }
            }
          }
        }
      }
      frame True {
        n1177 = local write "Manual Humididty Reached"(TRUE ("Manual Humididty Reached")) -> ()
      }
    }
    n1178 = local read "Cap Live Image"() -> (w1080:bool)
    n1179 = local read "SCAR MEASURMENT"() -> (w1083:enum32{"Auto Scar", "Manual Scar"})
    n1180 = Equal?(x=w1083, y=enum32{"Auto Scar", "Manual Scar"}."Manual Scar" ("SCAR MEASURMENT")) -> (x = y?=w1081:bool)
    n1181 = And(x=w1081, y=w1080) -> (x .and. y?=w1079:bool)
    n1182 = Wait (ms)(milliseconds to wait=u32 250) -> ()  [unwired: 1 out]
    n1183 = case shown="True" w1079 {
      selector: w1079 -> [_ w1402]
      frame False {
      }
      frame True {
        n1184 = stacked-sequence {
          tunnel: [_ _ _ w1421 _] -> _
          tunnel: w1402 -> [_ _ _ _ w1428]
          frame #0 {
            w1403 = 0.0
            n1185 = local write "Major Axis"(w1403) -> ()
            n1186 = local write "Minor Axis"(w1403) -> ()
            n1187 = local write "Average"(w1403) -> ()
          }
          frame #1 {
            n1188 = call "CAMERA LIVE FEED FGV.vi"("Enum - Menu"=CAMERA_LIVE_FEED_ENUM."CAMERA MINIMIZE") -> ()  [unwired: 9 in, 2 out]
          }
          frame #2 {
            n1189 = local read "Magnification len live scar"() -> (w1407:string)
            n1190 = case shown="\"10x\", Default" w1407 {
              tunnel: ["_10x" "_5x"] -> w1406
              frame "10x", Default {
              }
              frame "5x" {
              }
            }
            n1191 = local read "FILE 3"() -> (w1413:string)
            n1192 = call <vilib>:"Trim Whitespace.vi"("string"="C:\\LAB-IQ\\images\\") -> ("trimmed string"=w1415:string)  [unwired: 1 in]
            n1193 = String To Path(string=w1415) -> (path=w1414:path)
            n1194 = Concatenate Strings(w1413, w1406, ".png" ("string")) -> (w1412:string)
            n1195 = Build Path(base path=w1414, name or relative path=w1412) -> (appended path=w1411:path)
            n1196 = Path To String(path=w1411) -> (string=w1410:string)
            n1197 = call "CAMERA LIVE FEED FGV.vi"("Enum - Menu"=CAMERA_LIVE_FEED_ENUM."CAMERA SAVE", "Image Path"=w1410) -> ("error out"=w1408:errorcluster)  [unwired: 8 in, 1 out]
            n1198 = case shown="No Error" w1408 {
              frame No Error {
                n1199 = One Button Dialog(message="Image saved successfully") -> ()  [unwired: 1 in, 1 out]
              }
              frame Error {
              }
            }
          }
          frame #3 {
            n1200 = call "LIST FILE NAMES.vi"() -> ("error out"=w1423:errorcluster, "filenames"=w1420:string[])  [unwired: 10 in]
            n1201 = call "IMAGE ANALYSIS.vi"("Enum"=POST_ANALYSIS_ENUM."SHOW UI", "error in"=w1423) -> ("error out"=w1421:errorcluster)  [unwired: 8 in, 1 out]
            n1202 = property on="Test File List :" class="CmbBox"("Strings[]"=w1420) -> ()  [unwired: 2 in, 2 out]
          }
          frame #4 {
            (unwired) T25."Report" ("Main Dashboard Buttons")
            (unwired) T27."Report" ("Main Dashboard Buttons")
            n1203 = Not(x=w1428) -> (.not. x?=w1427:bool)
            n1204 = local write "Zoom Factore"(0.0 ("Zoom Factore")) -> ()
            n1205 = local write "Cap Live Image"(w1427) -> ()
            n1206 = local write "Main Tab"(T2."Adv Scar Report" ("Main Tab")) -> ()
            n1207 = property on="Cap Live Image" class="Bool (strict)"("BoolText.Text"="Capture Image" ("Boolean Text.Text")) -> ()  [unwired: 2 in, 2 out]
            n1208 = local write "Main Dashboard Buttons"(T1."Report" ("Main Dashboard Buttons")) -> ()
          }
        }
      }
    }
    n1209 = local read "change Gain"() -> (w1063:bool)
    n1210 = local read "Back Square"() -> (w1062:bool)
    n1211 = case shown="True" w1063 {
      selector: w1063 -> [_ w1107]
      frame False {
      }
      frame True {
        n1212 = stacked-sequence {
          tunnel: w1107 -> [_ w1115]
          frame #0 {
            n1213 = local read "Actual (µm)"() -> (w1111:dbl)
            n1214 = local read "Pixel Value"() -> (w1110:dbl)
            n1215 = local read "Magnification :"() -> (w1109:string)
            n1216 = Divide(x=w1111, y=w1110) -> (x/y=w1108:dbl)
            n1217 = case shown="\"10x\"" w1109 {
              tunnel: w1108 -> [w1112 w1113]
              frame "10x" {
                n1218 = local write "10x Gain"(w1112) -> ()
              }
              frame "5x", Default {
                n1219 = local write "5x Gain"(w1113) -> ()
              }
            }
          }
          frame #1 {
            n1220 = Not(x=w1115) -> (.not. x?=w1114:bool)
            n1221 = local write "change Gain"(w1114) -> ()
          }
        }
      }
    }
    n1222 = case shown="True" w1062 {
      selector: w1062 -> [_ w1105]
      frame False {
      }
      frame True {
        n1223 = Not(x=w1105) -> (.not. x?=w1104:bool)
        n1224 = local write "Back Square"(w1104) -> ()
        n1225 = local write "Calibration Tab"(enum32{"Measrument", "Calibrate"}."Measrument" ("Calibration Tab")) -> ()
      }
    }
    n1226 = local read "Rectangle Tool"() -> (w1074:bool)
    n1227 = local read "Clear ROI Tool"() -> (w1073:bool)
    n1228 = local read "Open Image"() -> (w1078:bool)
    n1229 = local read "line tool"() -> (w1075:bool)
    n1230 = local read "OUT"() -> (w1076:bool)
    n1231 = local read "In"() -> (w1077:bool)
    n1232 = case shown="True" w1078 {
      selector: w1078 -> [_ w1388]
      tunnel: [w1379 w1390] -> _
      tunnel: w1068 -> [w1379 w1389]
      frame False {
      }
      frame True {
        w1383 = "_5x" ("regular expression")
        n1233 = Not(x=w1388) -> (.not. x?=w1387:bool)
        n1234 = local write "Open Image"(w1387) -> ()
        n1235 = call "IMAGE ANALYSIS.vi"("Enum"=POST_ANALYSIS_ENUM."HIDE UI", "error in"=w1389) -> ("error out"=w1397:errorcluster)  [unwired: 8 in, 1 out]
        n1236 = call <vilib>:"Clear Errors.vi"("error in (no error)"=w1397) -> ("error out"=w1380:errorcluster)  [unwired: 5 in, 1 out]
        n1237 = call "File Dialog"("start path"=path "C:/LAB-IQ/images", "error in"=w1380) -> ("selected path"=w1382:path, "error out"=w1395:errorcluster)  [unwired: 10 in, 2 out]
        "Image path  2" <- w1382
        n1238 = call <vilib>:"Clear Errors.vi"("error in (no error)"=w1395) -> ("error out"=w1394:errorcluster)  [unwired: 5 in, 1 out]
        n1239 = call "IMAGE ANALYSIS.vi"("Enum"=POST_ANALYSIS_ENUM."OPEN FILE", "error in"=w1394, "File Path"=w1382) -> ("error out"=w1393:errorcluster)  [unwired: 7 in, 1 out]
        n1240 = call <vilib>:"Clear Errors.vi"("error in (no error)"=w1393) -> ("error out"=w1392:errorcluster)  [unwired: 5 in, 1 out]
        n1241 = call "IMAGE ANALYSIS.vi"("Enum"=POST_ANALYSIS_ENUM."SHOW UI", "error in"=w1392) -> ("error out"=w1390:errorcluster)  [unwired: 8 in, 1 out]
        n1242 = local write "Zoom Factore"(100.0 ("Zoom Factore")) -> ()
        n1243 = Strip Path(path=w1382) -> (name=w1385:string)  [unwired: 1 out]
        n1244 = Match Pattern(string=w1385, regular expression=w1383) -> (match substring=w1384:string)  [unwired: 1 in, 3 out]
        n1245 = Equal?(x=w1384, y=w1383) -> (x = y?=w1381:bool)
        n1246 = case shown="False" w1381 {
          frame False {
            n1247 = local write "Magnification :"("10x" ("Magnification :")) -> ()
          }
          frame True {
            n1248 = local write "Magnification :"("5x" ("Magnification :")) -> ()
          }
        }
      }
    }
    n1249 = case shown="True" w1076 {
      selector: w1076 -> [_ w1364]
      tunnel: w1068 -> [w1361 w1369]
      tunnel: [w1361 w1363] -> _
      frame False {
      }
      frame True {
        n1250 = Not(x=w1364) -> (.not. x?=w1362:bool)
        n1251 = local read "Zoom Factore"() -> (w1367:dbl)
        n1252 = local write "OUT"(w1362) -> ()
        n1253 = call "IMAGE ANALYSIS.vi"("Enum"=POST_ANALYSIS_ENUM."ZOOM OUT", "error in"=w1369) -> ("error out"=w1363:errorcluster)  [unwired: 8 in, 1 out]
        n1254 = Divide(x=w1367, y=1.2) -> (x/y=w1365:dbl)
        n1255 = local write "Zoom Factore"(w1365) -> ()
      }
    }
    n1256 = case shown="True" w1077 {
      selector: w1077 -> [_ w1373]
      tunnel: w1068 -> [w1370 w1378]
      tunnel: [w1370 w1371] -> _
      frame False {
      }
      frame True {
        n1257 = Not(x=w1373) -> (.not. x?=w1372:bool)
        n1258 = local read "Zoom Factore"() -> (w1376:dbl)
        n1259 = local write "In"(w1372) -> ()
        n1260 = call "IMAGE ANALYSIS.vi"("Enum"=POST_ANALYSIS_ENUM."ZOOM IN", "error in"=w1378) -> ("error out"=w1371:errorcluster)  [unwired: 8 in, 1 out]
        n1261 = Multiply(x=w1376, y=1.2) -> (x*y=w1374:dbl)
        n1262 = local write "Zoom Factore"(w1374) -> ()
      }
    }
    n1263 = case shown="True" w1073 {
      selector: w1073 -> [_ w1345]
      tunnel: w1068 -> [w1343 w1347]
      tunnel: [w1343 w1346] -> _
      frame False {
      }
      frame True {
        n1264 = Not(x=w1345) -> (.not. x?=w1344:bool)
        n1265 = local write "Clear ROI Tool"(w1344) -> ()
        n1266 = call "IMAGE ANALYSIS.vi"("Enum"=POST_ANALYSIS_ENUM."CLEAR ROI", "error in"=w1347) -> ("error out"=w1346:errorcluster)  [unwired: 8 in, 1 out]
      }
    }
    n1267 = case shown="True" w1075 {
      selector: w1075 -> [_ w1357]
      tunnel: w1068 -> [w1355 w1360]
      tunnel: [w1355 w1358] -> _
      frame False {
      }
      frame True {
        n1268 = Not(x=w1357) -> (.not. x?=w1356:bool)
        n1269 = local write "line tool"(w1356) -> ()
        n1270 = call "IMAGE ANALYSIS.vi"("Enum"=POST_ANALYSIS_ENUM."DRAW LINE", "error in"=w1360) -> ("error out"=w1358:errorcluster)  [unwired: 8 in, 1 out]
      }
    }
    n1271 = case shown="True" w1074 {
      selector: w1074 -> [_ w1351]
      tunnel: w1068 -> [w1349 w1353]
      tunnel: [w1349 w1352] -> _
      frame False {
      }
      frame True {
        n1272 = Not(x=w1351) -> (.not. x?=w1350:bool)
        n1273 = local write "Rectangle Tool"(w1350) -> ()
        n1274 = call "IMAGE ANALYSIS.vi"("Enum"=POST_ANALYSIS_ENUM."DRAW REC", "error in"=w1353) -> ("error out"=w1352:errorcluster)  [unwired: 8 in, 1 out]
      }
    }
    n1275 = local read "SCAR MEASURMENT"() -> (w1061:enum32{"Auto Scar", "Manual Scar"})
    n1276 = local read "Fit to Screen Tool"() -> (w1070:bool)
    n1277 = local read "Resize Tool"() -> (w1069:bool)
    n1278 = case shown="\"Manual Scar\", Default" w1061 {
      frame "Auto Scar" {
        n1279 = property on="Cap Live Image" class="Bool (strict)"("BoolText.Text"="Report" ("Boolean Text.Text")) -> ()  [unwired: 2 in, 2 out]
      }
      frame "Manual Scar", Default {
        n1280 = property on="Cap Live Image" class="Bool (strict)"("BoolText.Text"="Save Image" ("Boolean Text.Text")) -> ()  [unwired: 2 in, 2 out]
      }
    }
    n1281 = local read "ROI Color Tool"() -> (w1071:bool)
    n1282 = local read "Pan Tool"() -> (w1072:bool)
    n1283 = case shown="True" w1072 {
      selector: w1072 -> [_ w1339]
      tunnel: w1068 -> [w1337 w1341]
      tunnel: [w1337 w1340] -> _
      frame False {
      }
      frame True {
        n1284 = Not(x=w1339) -> (.not. x?=w1338:bool)
        n1285 = call "IMAGE ANALYSIS.vi"("Enum"=POST_ANALYSIS_ENUM."PAN", "error in"=w1341) -> ("error out"=w1340:errorcluster)  [unwired: 8 in, 1 out]
        n1286 = local write "Pan Tool"(w1338) -> ()
      }
    }
    n1287 = case shown="True" w1069 {
      selector: w1069 -> [_ w1323]
      tunnel: w1068 -> [w1318 w1320]
      tunnel: [w1318 w1319] -> _
      frame False {
      }
      frame True {
        n1288 = Not(x=w1323) -> (.not. x?=w1322:bool)
        n1289 = local write "Resize Tool"(w1322) -> ()
        n1290 = call "IMAGE ANALYSIS.vi"("Enum"=POST_ANALYSIS_ENUM."RESIZE MODE", "error in"=w1320) -> ("error out"=w1319:errorcluster)  [unwired: 8 in, 1 out]
      }
    }
    n1291 = case shown="True" w1070 {
      selector: w1070 -> [_ w1328]
      tunnel: [w1324 w1329] -> _
      tunnel: w1068 -> [w1324 w1327]
      frame False {
      }
      frame True {
        n1292 = Not(x=w1328) -> (.not. x?=w1326:bool)
        n1293 = local write "Zoom Factore"(100.0 ("Zoom Factore")) -> ()
        n1294 = local write "Fit to Screen Tool"(w1326) -> ()
        n1295 = call "IMAGE ANALYSIS.vi"("Enum"=POST_ANALYSIS_ENUM."FIT", "error in"=w1327) -> ("error out"=w1329:errorcluster)  [unwired: 8 in, 1 out]
      }
    }
    n1296 = case shown="True" w1071 {
      selector: w1071 -> [_ w1334]
      tunnel: [w1331 w1335] -> _
      tunnel: w1068 -> [w1331 w1332]
      frame False {
      }
      frame True {
        n1297 = Not(x=w1334) -> (.not. x?=w1333:bool)
        n1298 = local write "ROI Color Tool"(w1333) -> ()
        n1299 = call "IMAGE ANALYSIS.vi"("Enum"=POST_ANALYSIS_ENUM."SET ROI COLOR", "error in"=w1332) -> ("error out"=w1335:errorcluster)  [unwired: 8 in, 1 out]
      }
    }
    n1300 = local read "Quit"() -> (w1085:bool)
  }
  n1301 = while {
    stop <- w1430 stop-if-true
    n1302 = local read "Image Path"() -> (w1433:path)
    n1303 = local read "Print 3"() -> (w1436:bool)
    n1304 = Equal?(x=w1433, y=path "") -> (x = y?=w1432:bool)
    n1305 = Not(x=w1432) -> (.not. x?=w1431:bool)
    n1306 = property on="Print 3" class="Bool (strict)"("Visible"=w1431) -> ()  [unwired: 2 in, 2 out]
    n1307 = case shown="True" w1436 {
      frame False {
        n1308 = local write "Rd"(TRUE ("Boolean 7")) -> ()
      }
      frame True {
        n1309 = flat-sequence {
          tunnel: [w1476] -> w1444
          tunnel: [w1463] -> w1442
          tunnel: [w1473] -> w1438
          tunnel: w1444 -> [w1485]
          tunnel: [w1485] -> w1443
          tunnel: w1442 -> [w1484]
          tunnel: [w1484] -> w1441
          tunnel: [w1482] -> w1440
          tunnel: [w1481] -> w1439
          tunnel: w1438 -> [w1481]
          tunnel: w1443 -> [w1487]
          tunnel: w1441 -> [w1488]
          tunnel: w1440 -> [_]
          tunnel: w1439 -> [w1486]
          frame #0 {
            n1310 = case shown="True" "Rd" {
              frame False {
              }
              frame True {
                n1311 = while {
                  tunnel: "abcdefABCDEF" ("string 2") -> [w1455]
                  shift-right: [w1453] -> w1447
                  shift-left: "" -> [w1452]
                  i -> [w1462]
                  stop <- w1461 stop-if-true
                  n1312 = Random Number (0-1)() -> (number: 0 to 1=w1456:dbl)
                  n1313 = Multiply(x=w1456, y=62.0) -> (x*y=w1458:dbl)
                  n1314 = Decrement(x="Length 2") -> (x-1=w1451:i16)
                  n1315 = To Word Integer(number=w1458) -> (16bit integer=w1459:i16)
                  n1316 = String Subset(string=w1455, offset (0)=w1459, length (rest)=1 ("length (rest)")) -> (substring=w1454:string)
                  n1317 = Greater Or Equal?(x=w1462, y=w1451) -> (x >= y?=w1461:bool)
                  n1318 = Concatenate Strings(w1454, w1452) -> (w1453:string)
                }
                "String 10" <- w1447
                n1319 = local write "Rd"(FALSE ("Boolean 7")) -> ()
              }
            }
          }
          frame #1 {
            w1474 = "_resized.jpg" ("command line")
            (unwired) ".jpg -resize 320x240 " ("string")
            (unwired) "Choose an Image File" ("prompt")
            # "-resize 1798x425"
            n1320 = local read "Image Path"() -> (w1468:path)
            n1321 = Strip Path(path=w1468) -> (stripped path=w1463:path, name=w1464:string)
            n1322 = Match Pattern(string=w1464, regular expression=".jpg") -> (before substring=→"before substring 2":string, after substring=→"after substring":string)  [unwired: 1 in, 2 out]
            n1323 = Match Pattern(string=w1464, regular expression="\\") -> (before substring=w1470:string)  [unwired: 1 in, 3 out]
            n1324 = Match Pattern(string=w1470, regular expression=".jpg") -> (before substring=w1469:string)  [unwired: 1 in, 3 out]
            n1325 = Concatenate Strings("cmd /c convert " ("string"), w1469, ".jpg -resize 320x240  " ("command line"), w1469, w1474) -> (w1477:string)
            n1326 = call <vilib>:"System Exec.vi"("run minimized? (F)"=TRUE, "wait until completion? (T)"=TRUE, "working directory"=w1463, "command line"=w1477) -> ("error out"=w1476:errorcluster)  [unwired: 4 in, 3 out]
            "error out 2" <- w1476
            n1327 = Concatenate Strings(w1469, w1474) -> (w1473:string)
          }
          frame #2 {
            n1328 = Wait (ms)(milliseconds to wait=u32 2000 ("millisecond timer value")) -> (millisecond timer value=w1482:u32)
          }
          frame #3 {
            n1329 = case shown="No Error" w1487 {
              tunnel: w1488 -> [w1491 _]
              tunnel: w1486 -> [w1489 _]
              frame No Error {
                (unwired) ".jpg" ("string")
                n1330 = Path To String(path=w1491) -> (string=w1495:string)
                n1331 = Concatenate Strings(w1495, "\\" ("string"), w1489) -> (w1494:string)
                n1332 = String To Path(string=w1494) -> (path=w1493:path)
                n1333 = call <vilib>:"Read JPEG File.vi"("path to JPEG file"=w1493) -> ("image data"=w1497:T16)  [unwired: 8 in, 2 out]
                "image data" <- w1497
                n1334 = local write "Print 3"(FALSE ("Print 2")) -> ()
                n1335 = call <vilib>:"Draw Flattened Pixmap.vi"("image data"=w1497) -> ("new picture"=→"new picture":picture)  [unwired: 8 in]
              }
              frame Error {
              }
            }
          }
        }
      }
    }
    n1336 = Wait (ms)(milliseconds to wait=u32 20 ("millisecond timer value")) -> ()  [unwired: 1 out]
    n1337 = local read "Quit"() -> (w1430:bool)